vi "AVI saves prototyping-RGB.vi"() -> ()   [LabVIEW 2017]
uses:
  <vilib>/vision/Image Controls.llb/IMAQ Image.ctl
  <vilib>/vision/Avi.llb/IMAQ AVI2 Codec Path.ctl
  Typedefs/Frame Size.ctl
  <vilib>/vision/NI_Vision_Development_Module.lvlib
panel:
  out "size(s) 6":i32[](array[numeric])
  out "size(s) 5":i32[](array[numeric])
  out "OK 2":bool
  out "Image 3":T1(plugin-control)
  out "Image 2":T1(plugin-control)
  out "size(s) 4":i32[](array[numeric])
  out "Image Pixels (U32)":u32[][](array[numeric])
  out "max value 3":i16
  out "max value 2":i16
  out "size(s) 3":i32[](array[numeric])
  out "Image Pixels (I16) 2":u32[][][](array[numeric])
  out "Image Pixels (I16)":i16[][][](array[numeric])
  out "Read time (ms)":u32
  out "Average frame write frequency":dbl
  out "Write time (ms)":u32
  out "size(s) 2":i32[](array[numeric])
  out "size(s)":i32[](array[numeric])
  in  "GreenImageArray":T1[](array[typedef])=["remote image 0000000015F6793C", "remote image 0000000015F679A4", "remote image 0000000015F67A0C", "remote image 0000000015F67A74", "remote image 0000000015F67ADC", "remote image 0000000015F67B44", "remote image 0000000015F67BAC"]
  out "x = y?":bool[][][](array[boolean])
  out "OK":bool
  out "Image":T1(plugin-control)
  out "output array":u32[][](array[numeric])
  out "# of frames written":i32
  out "Codec Used":string
  in  "Frames to write":i32=7
  in  "stop":bool
  in  "Quality":i32=750
  in  "Codex index":i32
  out "Codec Names":string[](array[string])
  in  "AVI File Path":path=path "C:/Users/Teo/Desktop/test.avi"
  in  "Rate (Hz)":u32=10
  # "Frame data saved in these\n7 image/frame references"
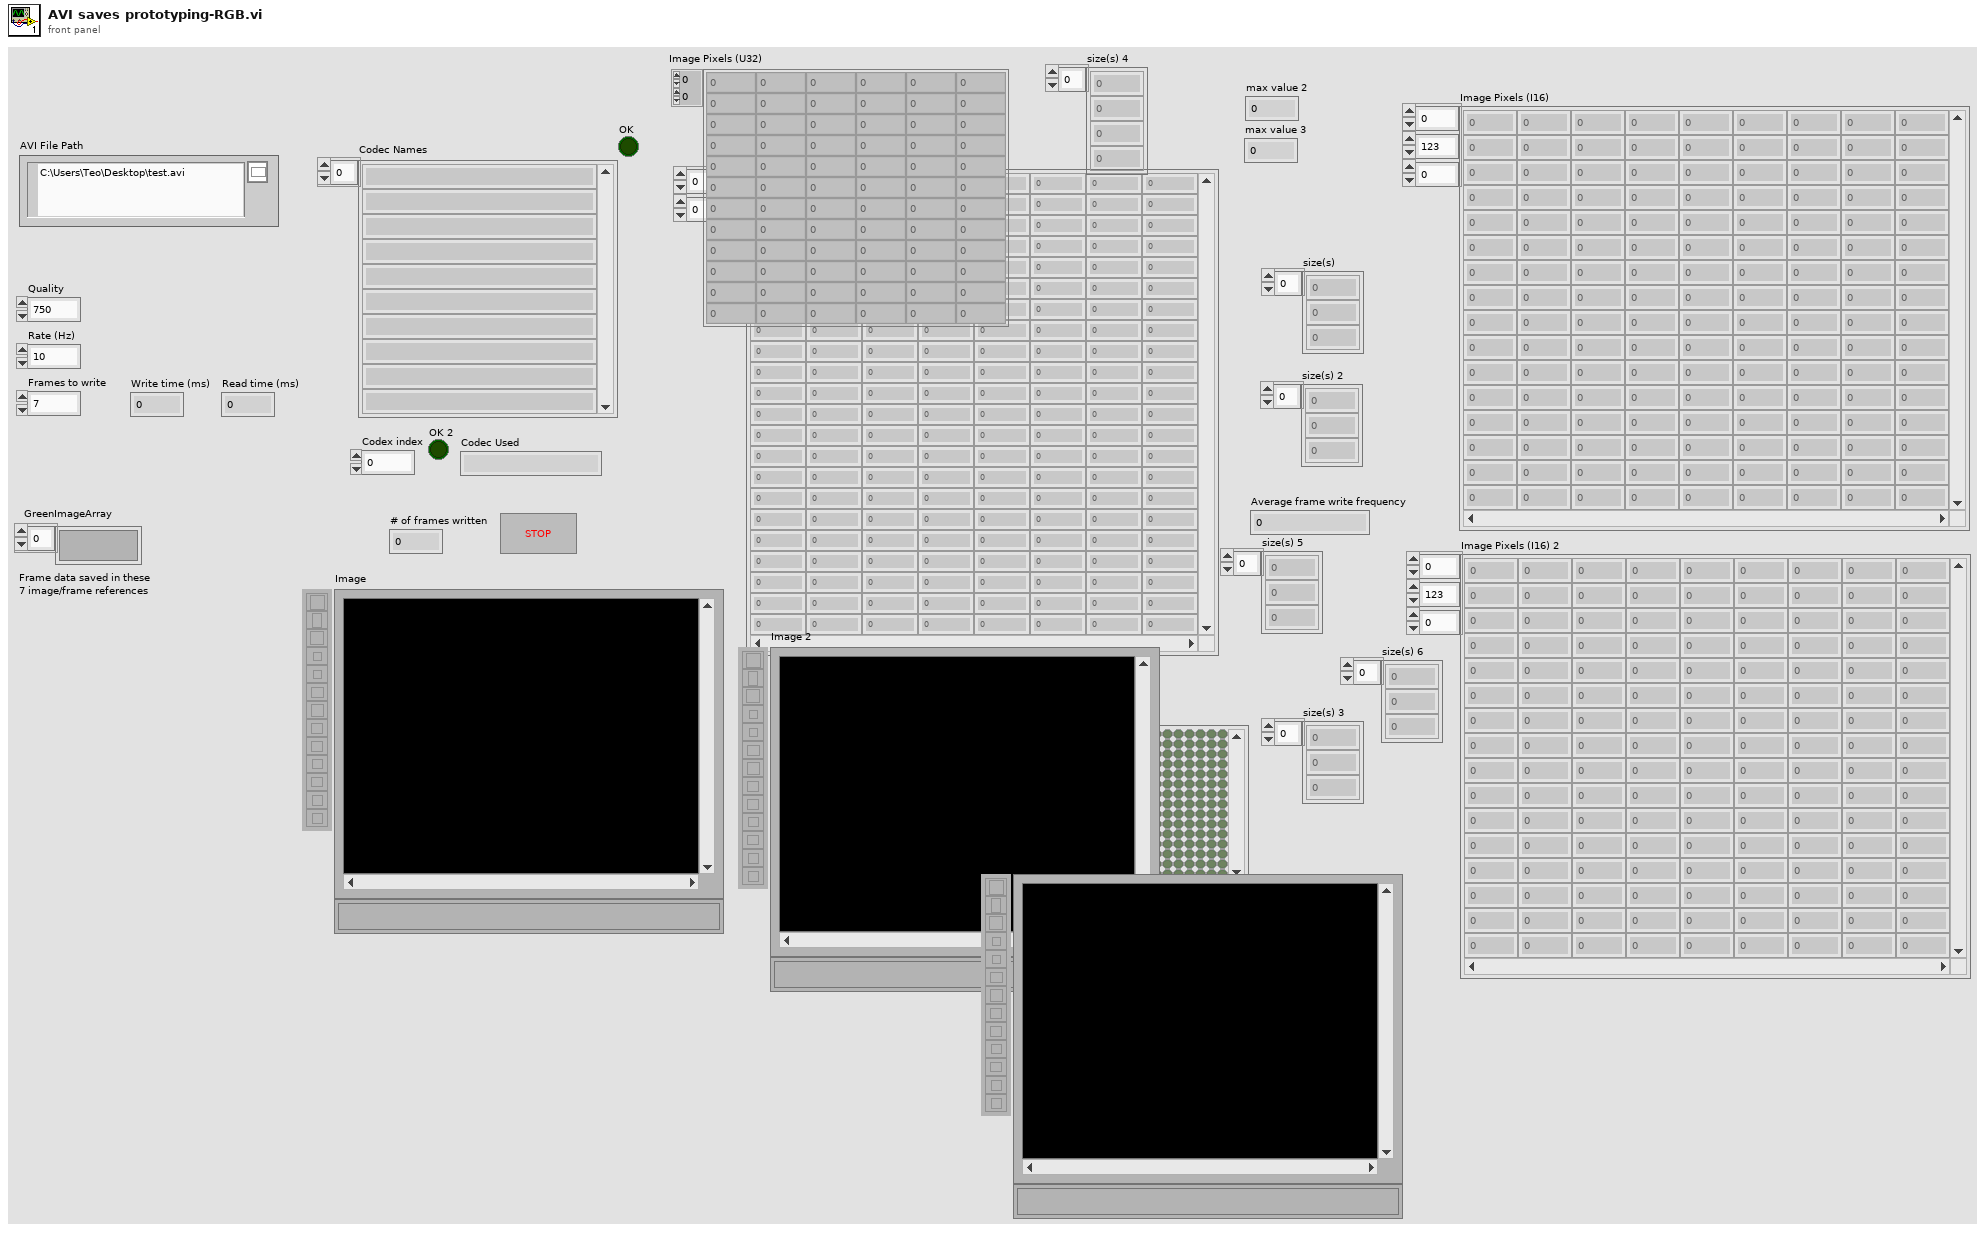
[diagram p1: front panel]
types:
  T1 = typedef "IMAQ Image.ctl" = refnum<image>
  T2 = typedef "Image Type" = u32
  T3 = typedef "IMAQ AVI2 Codec Path.ctl" = u32
  T4 = typedef "Color (U64)" = cluster{"Plane 3 (Blue)":u16, "Plane 2 (Green)":u16, "Plane 1 (Red)":u16, "Plane 4 (alpha)":u16}
  T5 = typedef "IMAQ AVI2 Refnum.ctl" = refnum<k20>
  T6 = typedef "Frame Size.ctl" = u16
  T7 = cluster{"Red (or Hue) value":u8, "Green (or Sat) value":u8, "Blue (or Light or Val) value":u8}[][]
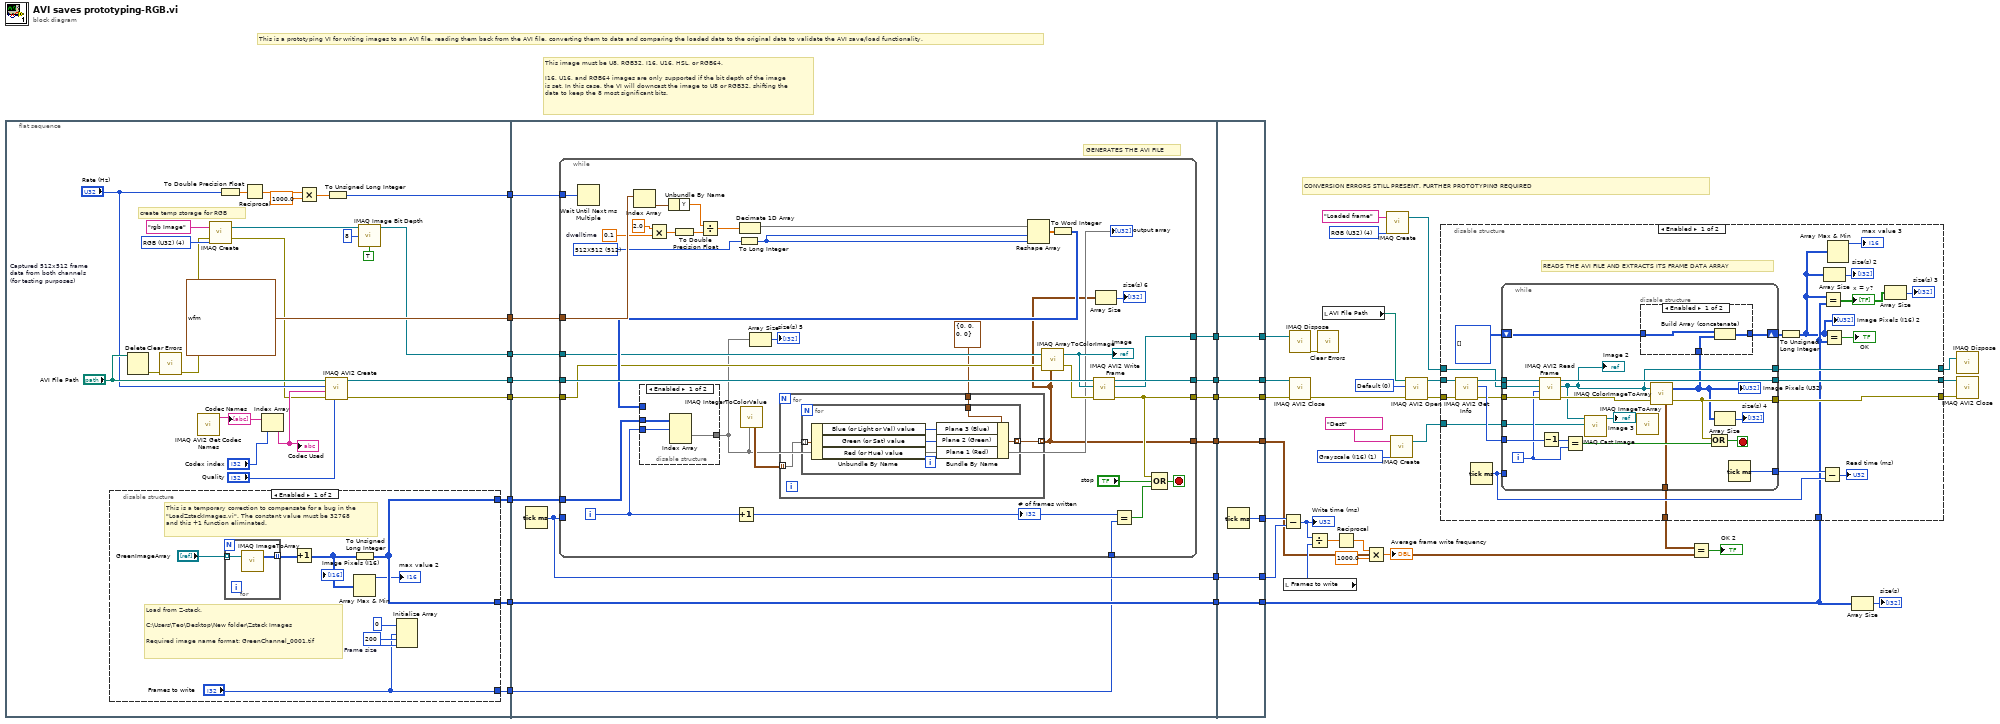
[diagram p0: block diagram]
diagram:
  w6 = T2 1 items=["Grayscale (U8)", "Grayscale (I16)", "Grayscale (SGL)", "Complex (CSG)", "RGB (U32)", "HSL (U32)", "RGB (U64)", "Grayscale (U16)"] ("Image Type")
  w37 = T2 4 items=["Grayscale (U8)", "Grayscale (I16)", "Grayscale (SGL)", "Complex (CSG)", "RGB (U32)", "HSL (U32)", "RGB (U64)", "Grayscale (U16)"] ("Image Type")
  w42 = T3 0 items=["Default", "System", "Built in Vision"] ("Codec Source")
  # "CONVERSION ERRORS STILL PRESENT. FURTHER PROTOTYPING REQUIRED"
  # "This is a prototyping VI for writing images to an AVI file, reading them back from the AVI file, converting them to data and comparing the loaded data to the original data to validate the AVI save/load functionality."
  # "This image must be U8, RGB32, I16, U16, HSL, or RGB64. \n\nI16, U16, and RGB64 images are only supported if the bit depth of the image is set. In this case, the VI will downcast the image to U8 or RGB32, shifting the data to keep the 8 most significant bits."
  n1 = flat-sequence {
    tunnel: [w71] -> w31
    tunnel: [w65] -> w30
    tunnel: [w64] -> w29
    tunnel: [w62] -> w28
    tunnel: [w59] -> w27
    tunnel: [w49] -> w26
    tunnel: [w53] -> w25
    tunnel: [w52] -> w8
    tunnel: w31 -> [w92]
    tunnel: w30 -> [w90]
    tunnel: w29 -> [w89]
    tunnel: w28 -> [w91]
    tunnel: w27 -> [w87]
    tunnel: w26 -> [w88]
    tunnel: w25 -> [w93]
    tunnel: [w90] -> w21
    tunnel: [w93] -> w20
    tunnel: [w86] -> w19
    tunnel: [w85] -> w18
    tunnel: [w84] -> w16
    tunnel: w8 -> [w83]
    tunnel: [w82] -> w4
    tunnel: [w145] -> w22
    tunnel: [w146] -> w23
    tunnel: [w147] -> w33
    tunnel: [w148] -> w24
    tunnel: w21 -> [w148]
    tunnel: w20 -> [w147]
    tunnel: w19 -> [w146]
    tunnel: w18 -> [w145]
    tunnel: [w144] -> w17
    tunnel: w16 -> [w143]
    tunnel: [w143] -> w15
    tunnel: [w142] -> w1
    tunnel: w4 -> [w142]
    frame #0 {
      w61 = T2 4 items=["Grayscale (U8)", "Grayscale (I16)", "Grayscale (SGL)", "Complex (CSG)", "RGB (U32)", "HSL (U32)", "RGB (U64)", "Grayscale (U16)"] ("Image Type")
      w71 = waveform(dbl)[] [{"t0"=timestamp(0 s since 1904-01-01), "dt"=1.0, "Y"=array[524288 elements]}]  # Captured 512x512 frame data from both channels (for testing purposes)
      # "create temp storage for RGB"
      n2 = disable-structure shown="Enabled" {
        disable-tunnel: [w74 _] -> w59
        disable-tunnel: [w74 _] -> w53
        disable-tunnel: ["Frames to write" _] -> w52
        frame Enabled {
          w78 = 200  # Frame size
          # "This is a temporary correction to compensate for a bug in the \"LoadZstackImages.vi\". The constant value must be 32768 and this +1 function eliminated."
          # "Load from Z-stack.\n\nC:\\Users\\Teo\\Desktop\\New folder\\Zstack Images\n\nRequired image name format: GreenChannel_0001.tif"
          n3 = for {
            tunnel: "GreenImageArray" -> [w81] mode=indexing
            tunnel: [w80] -> w75 mode=indexing
            n4 = call "IMAQ ImageToArray"("Image"=w81) -> ("Image Pixels (I16)"=w80:i16[][])  [unwired: 3 in, 4 out]
          }
          n5 = Increment(x=w75) -> (x+1=w73:i16[][][])
          "Image Pixels (I16)" <- w73
          n6 = Array Max & Min(array=w73) -> (max value=→"max value 2":i16)  [unwired: 3 out]
          n7 = To Unsigned Long Integer(number=w73) -> (unsigned 32bit integer=w74:u32[][][])
          n8 = Initialize Array(u32 0, "Frames to write", w78, w78) -> ()  [unwired: 1 out]
        }
        frame Disabled {
        }
      }
      n9 = Delete(path (use dialog)="AVI File Path") -> (error out=w57:errorcluster)  [unwired: 4 in, 2 out]
      n10 = call <vilib>:"Clear Errors.vi"("error in (no error)"=w57) -> ("error out"=w56:errorcluster)  [unwired: 5 in, 1 out]
      n11 = call "IMAQ AVI2 Get Codec Names"() -> ("Codec Names"=w67:string[])  [unwired: 10 in, 1 out]
      "Codec Names" <- w67
      n12 = call "IMAQ Create"("Image Name"="rgb Image", "Image Type"=w61, "error in (no error)"=w56) -> ("New Image"=w50:T1, "error out"=w46:errorcluster)  [unwired: 2 in]
      n13 = To Double Precision Float(number="Rate (Hz)") -> (double precision float=w63:dbl)
      n14 = Reciprocal(x=w63) -> (1/x=w70:dbl)
      n15 = Index Array(array=w67, index="Codex index") -> (element=w58:string)
      "Codec Used" <- w58
      n16 = Multiply(x=w70, y=1000.0) -> (x*y=w68:dbl)
      n17 = call "IMAQ AVI2 Create"("Quality"="Quality", "error in (no error)"=w46, "Codec"=w58, "Frames Per Second"="Rate (Hz)", "AVI Path"="AVI File Path") -> ("error out"=w64:errorcluster, "AVI Refnum"=w65:T5)  [unwired: 5 in]
      n18 = To Unsigned Long Integer(number=w68) -> (unsigned 32bit integer=w62:u32)
      n19 = call "IMAQ Image Bit Depth"("Image"=w50, "Bit Depth (0)"=u32 8, "Get/Set Bit Depth? (Set)"=TRUE) -> ("Image Out"=w49:T1)  [unwired: 10 in, 2 out]
    }
    frame #1 {
      # "GENERATES THE AVI FILE"
      n20 = Tick Count (ms)() -> (millisecond timer value=w84:u32)
      n21 = while {
        tunnel: w92 -> [w116]
        tunnel: w91 -> [w128]
        tunnel: w90 -> [w125]
        tunnel: w89 -> [w104]
        tunnel: [w124] -> _
        tunnel: [w123] -> w86
        tunnel: [w111] -> w85
        tunnel: w88 -> [w106]
        tunnel: w87 -> [w108]
        tunnel: w84 -> [_]
        tunnel: w83 -> [w101]
        tunnel: [w94] -> w82
        i -> [w98]
        stop <- w127 stop-if-true
        w115 = 0.1  # dwelltime
        w113 = T6 512 items=["20X20"=0, "100X100"=100, "128X128"=128, "200X200"=200, "256X256"=256, "512X512"=512] ("Frame Size")
        n22 = Wait Until Next ms Multiple(millisecond multiple=w128) -> ()  [unwired: 1 out]
        n23 = Index Array(array=w116) -> (element=w121:waveform(dbl))  [unwired: 1 in]
        n24 = Multiply(x=2.0, y=w115) -> (x*y=w119:dbl)
        n25 = Unbundle By Name ("Get Waveform Components")(w121) -> ("Y"=w118:dbl[])
        n26 = To Double Precision Float(number=w119) -> (double precision float=w122:dbl)
        n27 = Divide(x=w118, y=w122) -> (x/y=w117:dbl[])
        n28 = Increment(x=w98) -> (x+1=w102:i32)
        "# of frames written" <- w102
        n29 = To Long Integer(number=w113) -> (32bit integer=w112:i32)
        n30 = Decimate 1D Array(w117) -> (w114:dbl[])  [unwired: 1 out]
        n31 = Reshape Array(w114, w112, w112) -> (w110:dbl[][])
        n32 = To Word Integer(number=w110) -> (16bit integer=w107:i16[][])
        n33 = disable-structure shown="Enabled" {
          disable-tunnel: w108 -> [w140 _]
          disable-tunnel: w98 -> [w139 _]
          disable-tunnel: [w138 w141] -> w95
          disable-tunnel: w107 -> [_ w141]
          frame Enabled {
            n34 = Index Array(array=w140, index (dim 0)=w139) -> (element=w138:u32[][])  [unwired: 2 in]
          }
          frame Disabled {
          }
        }
        "output array" <- w95
        n35 = call "IMAQ IntegerToColorValue"("2D U32 array"=w95) -> ("2D Color value array"=w100:T7)  [unwired: 4 in, 3 out]
        n36 = Array Size(array=w95) -> (size(s)=→"size(s) 5":i32[])
        n37 = for {
          tunnel: w100 -> [w131] mode=indexing
          tunnel: T4 {"Plane 3 (Blue)"=0, "Plane 2 (Green)"=0, "Plane 1 (Red)"=0, "Plane 4 (alpha)"=0} ("Color (U64)") -> [w130]
          tunnel: [w129] -> w94 mode=indexing
          n38 = for {
            tunnel: w131 -> [w136] mode=indexing
            tunnel: w130 -> [w137]
            tunnel: [w132] -> w129 mode=indexing
            n39 = Unbundle By Name(w136) -> ("Blue (or Light or Val) value"=w135:u8, "Green (or Sat) value"=w134:u8, "Red (or Hue) value"=w133:u8)
            n40 = Bundle By Name(cluster=w137, "Plane 3 (Blue)"=w135, "Plane 2 (Green)"=w134, "Plane 1 (Red)"=w133) -> (w132:T4)
          }
        }
        n41 = call "IMAQ ArrayToColorImage"("Image"=w106, "Image Pixels (U64)"=w94, "error in (no error)"=w104) -> ("Image Out"=w105:T1, "error out"=w103:errorcluster)  [unwired: 1 in, 1 out]
        "Image" <- w105
        n42 = call "IMAQ AVI2 Write Frame"("error in (no error)"=w103, "Image"=w105, "AVI Refnum"=w125) -> ("error out"=w123:errorcluster, "Image Out (duplicate)"=w111:T1, "AVI Refnum (duplicate)"=w124:T5)  [unwired: 6 in]
        n43 = Array Size(array=w94) -> (size(s)=→"size(s) 6":i32[])
        n44 = Equal?(x=w102, y=w101) -> (x = y?=w109:bool)
        n45 = Compound Arithmetic op=OR(w123, "stop", w109) -> (w127:bool)
      }
    }
    frame #2 {
      n46 = Tick Count (ms)() -> (millisecond timer value=w144:u32)
    }
  }
  n47 = Subtract(x=w17, y=w15) -> (x-y=w14:u32)
  "Write time (ms)" <- w14
  n48 = local read "Frames to write"() -> (w13:i32)
  n49 = call "IMAQ Dispose"("Image"=w22) -> ("error out"=w34:errorcluster)  [unwired: 2 in, 3 out]
  n50 = call "IMAQ AVI2 Close"("error in (no error)"=w23, "AVI Refnum"=w24) -> ("error out"=w35:errorcluster)  [unwired: 9 in]
  n51 = Divide(x=w14, y=w13) -> (x/y=w11:dbl)
  n52 = call <vilib>:"Clear Errors.vi"("error in (no error)"=w34) -> ()  [unwired: 5 in, 2 out]
  n53 = local read "AVI File Path"() -> (w40:path)
  n54 = Reciprocal(x=w11) -> (1/x=w10:dbl)
  n55 = Multiply(x=w10, y=1000.0) -> (x*y=→"Average frame write frequency":dbl)
  n56 = call "IMAQ Create"("Image Name"="Loaded frame", "Image Type"=w37) -> ("New Image"=w36:T1)  [unwired: 3 in, 1 out]
  n57 = call "IMAQ Create"("Image Name"="Dest", "Image Type"=w6) -> ("New Image"=w5:T1)  [unwired: 3 in, 1 out]
  n58 = call "IMAQ AVI2 Open"("error in (no error)"=w35, "Codec Source"=w42, "AVI File Path"=w40) -> ("error out"=w39:errorcluster, "AVI Refnum"=w41:T5)  [unwired: 7 in]
  n59 = disable-structure shown="Enabled" {
    disable-tunnel: w33 -> [w156 _]
    disable-tunnel: w36 -> [w166 w195]
    disable-tunnel: w41 -> [w165 w197]
    disable-tunnel: w39 -> [w164 w196]
    disable-tunnel: [w162 w197] -> w45
    disable-tunnel: [w161 w196] -> w44
    disable-tunnel: [w163 w195] -> w43
    disable-tunnel: w5 -> [w150 _]
    disable-tunnel: [w149 _] -> w2
    frame Enabled {
      # "READS THE AVI FILE AND EXTRACTS ITS FRAME DATA ARRAY"
      n60 = call "IMAQ AVI2 Get Info"("error in (no error)"=w164, "AVI Refnum"=w165) -> ("error out"=w169:errorcluster, "Number of Frames"=w171:u32, "AVI Refnum (duplicate)"=w170:T5)  [unwired: 5 in, 2 out]
      n61 = Tick Count (ms)() -> (millisecond timer value=w157:u32)
      n62 = while {
        tunnel: w171 -> [w191]
        tunnel: w170 -> [w190]
        tunnel: w169 -> [w189]
        tunnel: w166 -> [w188]
        shift-right: [w187] -> w152
        shift-left: u32[][][] [] -> [w186]
        tunnel: [w175] -> w163
        tunnel: [w185] -> w162
        tunnel: [w182] -> w161
        tunnel: w157 -> [_]
        tunnel: [w178] -> w158
        tunnel: w150 -> [w176]
        tunnel: [w173] -> w149
        i -> [w179]
        stop <- w180 stop-if-true
        n63 = call "IMAQ AVI2 Read Frame"("error in (no error)"=w189, "Frame Number"=w179, "Image"=w188, "AVI Refnum"=w190) -> ("error out"=w183:errorcluster, "Image Out"=w175:T1, "AVI Refnum (duplicate)"=w185:T5)  [unwired: 5 in]
        "Image 2" <- w175
        n64 = Decrement(x=w191) -> (x-1=w184:u32)
        n65 = Equal?(x=w184, y=w179) -> (x = y?=w181:bool)
        n66 = call "IMAQ Cast Image"("Image Dst"=w176, "Image Src"=w175) -> ("Image Dst Out"=w174:T1)  [unwired: 8 in, 1 out]
        "Image 3" <- w174
        n67 = call "IMAQ ImageToArray"("Image"=w174) -> ()  [unwired: 3 in, 5 out]
        n68 = call "IMAQ ColorImageToArray"("Image"=w175, "error in (no error)"=w183) -> ("Image Pixels (U32)"=w172:u32[][], "error out"=w182:errorcluster, "Image Pixels (U64)"=w173:T4[][])  [unwired: 2 in]
        "Image Pixels (U32)" <- w172
        n69 = disable-structure shown="Enabled" {
          disable-tunnel: [w194 _] -> w187
          disable-tunnel: w186 -> [w193 _]
          disable-tunnel: w172 -> [w192 _]
          frame Enabled {
            n70 = Build Array (concatenate)(w193, w192) -> (w194:u32[][][])
          }
          frame Disabled {
          }
        }
        n71 = Compound Arithmetic op=OR(w182, w181) -> (w180:bool)
        n72 = Array Size(array=w172) -> (size(s)=→"size(s) 4":i32[])
        n73 = Tick Count (ms)() -> (millisecond timer value=w178:u32)
      }
      n74 = To Unsigned Long Integer(number=w152) -> (unsigned 32bit integer=w151:u32[][][])
      "Image Pixels (I16) 2" <- w151
      n75 = Subtract(x=w158, y=w157) -> (x-y=→"Read time (ms)":u32)
      n76 = Equal?(x=w151, y=w156) -> (x = y?=w154:bool[][][])
      "x = y?" <- w154
      n77 = Array Size(array=w151) -> (size(s)=→"size(s) 2":i32[])
      n78 = Equal?(x=w151, y=w156) -> (x = y?=→"OK":bool)
      n79 = Array Max & Min(array=w151) -> (max value=→"max value 3":u32)  [unwired: 3 out]
      n80 = Array Size(array=w154) -> (size(s)=→"size(s) 3":i32[])
    }
    frame Disabled {
    }
  }
  n81 = Equal?(x=w2, y=w1) -> (x = y?=→"OK 2":bool)
  n82 = Array Size(array=w33) -> (size(s)=→"size(s)":i32[])
  n83 = call "IMAQ Dispose"("Image"=w43) -> ()  [unwired: 2 in, 4 out]
  n84 = call "IMAQ AVI2 Close"("error in (no error)"=w44, "AVI Refnum"=w45) -> ()  [unwired: 9 in, 1 out]
